vi "Dresden R2R Sputter 03.02.2018 IY24.vi"() -> ()   [LabVIEW 2009] (continued)
                                n24398 = local write "Region"(w29818) -> ()
                                }
                                frame #1 {
                                n24399 = local write "Calculate_auto"(TRUE ("Calculate_auto")) -> ()
                                n24400 = Wait (ms)(milliseconds to wait=u32 1000) -> ()  [unwired: 1 out]
                                }
                                frame #2 {
                                n24401 = local write "Roll_side_select"(enum32{"Left to Right", "Right to Left"}."Left to Right" ("Roll_side_select")) -> ()
                                }
                                frame #3 {
                                n24402 = local write "Parameters_auto_set"(TRUE ("Parameters_auto_set")) -> ()
                                }
                                frame #4 {
                                n24403 = while {
                                i -> [w29834]
                                stop <- w29829 stop-if-true
                                n24404 = Greater?(x=w29834, y=1) -> (0:w29830:bool)
                                n24405 = Wait Until Next ms Multiple(millisecond multiple=u32 300) -> ()  [unwired: 1 out]
                                n24406 = local read "Parameters_auto_set"() -> (w29828:bool)
                                n24407 = case shown="False" w29828 {
                                tunnel: [TRUE FALSE] -> w29831
                                frame #0 {
                                }
                                frame #1 {
                                }
                                }
                                n24408 = Or(x=w29831, y=w29830) -> (x .or. y?=w29829:bool)
                                }
                                }
                                frame #5 {
                                n24409 = local read "R Tension Value"() -> (w29838:dbl)
                                n24410 = Wait (ms)(milliseconds to wait=u32 1000) -> ()  [unwired: 1 out]
                                n24411 = local write "TC1_set_value"(w29838) -> ()
                                }
                                frame #6 {
                                n24412 = local write "TC1_auto_set"(TRUE ("TC1_auto_set")) -> ()
                                }
                                frame #7 {
                                w29840 = u16 0 items=["1", "2", "3", "4"] ("Target Chamber Sensor")
                                n24413 = local write "Target Chamber Sensor"(w29840) -> ()
                                }
                                frame #8 {
                                n24414 = local read "Semi"() -> (w29841:bool)
                                n24415 = case shown="False" w29841 {
                                frame #0 {
                                # "Gas Flow"
                                n24416 = stacked-sequence {
                                frame #0 {
                                n24417 = stacked-sequence {
                                frame #0 {
                                n24418 = local read "Semi"() -> (w29842:bool)
                                n24419 = case shown="False" w29842 {
                                frame #0 {
                                n24420 = local write "Ar_sccm"(u16 200 ("Ar_sccm1_2")) -> ()
                                }
                                frame #1 {
                                }
                                }
                                }
                                frame #1 {
                                n24421 = local read "Semi"() -> (w29844:bool)
                                n24422 = case shown="False" w29844 {
                                frame #0 {
                                n24423 = local write "Mfc_Ar _set"(TRUE ("Mfc_Ar _1_2_set")) -> ()
                                }
                                frame #1 {
                                }
                                }
                                }
                                frame #2 {
                                n24424 = local read "Semi"() -> (w29846:bool)
                                n24425 = case shown="False" w29846 {
                                frame #0 {
                                n24426 = while {
                                i -> [w29850]
                                stop <- w29852 stop-if-true
                                n24427 = Greater?(x=w29850, y=50) -> (0:w29849:bool)
                                n24428 = local read "Semi"() -> (w29848:bool)
                                n24429 = case shown="True" w29848 {
                                tunnel: [FALSE TRUE] -> w29847
                                frame #0 {
                                n24430 = Wait Until Next ms Multiple(millisecond multiple=u32 200) -> ()  [unwired: 1 out]
                                }
                                frame #1 {
                                }
                                }
                                n24431 = Or(x=w29847, y=w29849) -> (x .or. y?=w29852:bool)
                                }
                                }
                                frame #1 {
                                }
                                }
                                }
                                frame #3 {
                                n24432 = local read "Semi"() -> (w29856:bool)
                                n24433 = case shown="False" w29856 {
                                frame #0 {
                                n24434 = local read "Ar_sccm_act 5"() -> (w29858:dbl)
                                n24435 = Greater?(x=w29858, y=1) -> (0:w29857:bool)
                                n24436 = case shown="False" w29857 {
                                frame #0 {
                                n24437 = local write "Ar_sccm"(u16 200 ("Ar_sccm1_2")) -> ()
                                }
                                frame #1 {
                                }
                                }
                                }
                                frame #1 {
                                }
                                }
                                }
                                frame #4 {
                                n24438 = local read "Semi"() -> (w29861:bool)
                                n24439 = case shown="False" w29861 {
                                frame #0 {
                                n24440 = local read "Ar_sccm_act 5"() -> (w29863:dbl)
                                n24441 = Greater?(x=w29863, y=1) -> (0:w29862:bool)
                                n24442 = case shown="False" w29862 {
                                frame #0 {
                                n24443 = while {
                                i -> [w29866]
                                stop <- w29870 stop-if-true
                                n24444 = Greater?(x=w29866, y=50) -> (0:w29865:bool)
                                n24445 = local read "Semi"() -> (w29869:bool)
                                n24446 = case shown="False" w29869 {
                                tunnel: [FALSE TRUE] -> w29868
                                frame #0 {
                                n24447 = Wait Until Next ms Multiple(millisecond multiple=u32 200) -> ()  [unwired: 1 out]
                                }
                                frame #1 {
                                }
                                }
                                n24448 = Or(x=w29868, y=w29865) -> (x .or. y?=w29870:bool)
                                }
                                }
                                frame #1 {
                                }
                                }
                                }
                                frame #1 {
                                }
                                }
                                }
                                frame #5 {
                                n24449 = local read "Semi"() -> (w29874:bool)
                                n24450 = case shown="False" w29874 {
                                frame #0 {
                                n24451 = local read "Ar_sccm_act 5"() -> (w29876:dbl)
                                n24452 = Greater?(x=w29876, y=1) -> (0:w29875:bool)
                                n24453 = case shown="False" w29875 {
                                frame #0 {
                                n24454 = local write "Semi"(TRUE ("Semi")) -> ()
                                n24455 = local write "Error Message"("Coating process cancelled.\nPlease check connections." ("Error Message")) -> ()
                                }
                                frame #1 {
                                }
                                }
                                }
                                frame #1 {
                                }
                                }
                                }
                                }
                                }
                                frame #1 {
                                n24456 = stacked-sequence {
                                frame #0 {
                                n24457 = local read "Semi"() -> (w29880:bool)
                                n24458 = case shown="False" w29880 {
                                frame #0 {
                                n24459 = local read "R_Single Microwave Power"() -> (w29882:dbl)
                                n24460 = Wait (ms)(milliseconds to wait=u32 200) -> ()  [unwired: 1 out]
                                n24461 = local write "Ch1_MW1"(w29882) -> ()
                                }
                                frame #1 {
                                }
                                }
                                }
                                frame #1 {
                                n24462 = local read "Semi"() -> (w29883:bool)
                                n24463 = case shown="False" w29883 {
                                frame #0 {
                                n24464 = local write "Ch1_MW1_set"(TRUE ("Microwave Power_auto_set")) -> ()
                                }
                                frame #1 {
                                }
                                }
                                }
                                frame #2 {
                                n24465 = local read "Semi"() -> (w29885:bool)
                                n24466 = case shown="False" w29885 {
                                frame #0 {
                                n24467 = Wait (ms)(milliseconds to wait=u32 1000) -> ()  [unwired: 1 out]
                                }
                                frame #1 {
                                }
                                }
                                }
                                frame #3 {
                                n24468 = local read "Semi"() -> (w29887:bool)
                                n24469 = case shown="False" w29887 {
                                frame #0 {
                                n24470 = local read "R_Single Microwave Power"() -> (w29889:dbl)
                                n24471 = Wait (ms)(milliseconds to wait=u32 200) -> ()  [unwired: 1 out]
                                n24472 = local write "Ch1_MW2"(w29889) -> ()
                                }
                                frame #1 {
                                }
                                }
                                }
                                frame #4 {
                                n24473 = local read "Semi"() -> (w29890:bool)
                                n24474 = case shown="False" w29890 {
                                frame #0 {
                                n24475 = local write "Ch1_MW2_set"(TRUE ("MW2_Power_set")) -> ()
                                }
                                frame #1 {
                                }
                                }
                                }
                                }
                                }
                                }
                                }
                                frame #1 {
                                }
                                }
                                }
                                frame #9 {
                                n24476 = local write "Start_roll"(TRUE ("Test_auto_start")) -> ()
                                n24477 = Wait (ms)(milliseconds to wait=u32 300) -> ()  [unwired: 1 out]
                                }
                                frame #10 {
                                n24478 = while {
                                stop <- w29895 stop-if-true
                                n24479 = local read "Actual Length"() -> (w29899:dbl)
                                n24480 = local read "Region"() -> (w29898:dbl)
                                n24481 = Greater Or Equal?(x=w29899, y=w29898) -> (x >= y?=w29896:bool)
                                n24482 = local read "Semi"() -> (w29897:bool)
                                n24483 = Or(x=w29896, y=w29897) -> (x .or. y?=w29895:bool)
                                n24484 = Wait Until Next ms Multiple(millisecond multiple=u32 300) -> ()  [unwired: 1 out]
                                }
                                }
                                frame #11 {
                                n24485 = local read "Semi"() -> (w29900:bool)
                                n24486 = case shown="False" w29900 {
                                frame #0 {
                                n24487 = Wait (ms)(milliseconds to wait=u32 1000) -> ()  [unwired: 1 out]
                                n24488 = local write "SMW15"(TRUE ("CMW12")) -> ()
                                }
                                frame #1 {
                                }
                                }
                                }
                                }
                                }
                                frame #1 {
                                }
                                }
                                }
                                frame #2 {
                                n24489 = local read "Semi"() -> (w29903:bool)
                                n24490 = case shown="False" w29903 {
                                frame #0 {
                                n24491 = stacked-sequence {
                                frame #0 {
                                n24492 = local read "R Maximum diameter"() -> (w29908:dbl)
                                n24493 = local read "R Minimum diameter"() -> (w29909:dbl)
                                n24494 = local read "R Web speed(cm/min)"() -> (w29906:dbl)
                                n24495 = local read "R _Total_length"() -> (w29904:dbl)
                                n24496 = local read "R Web thicness"() -> (w29907:dbl)
                                n24497 = Wait (ms)(milliseconds to wait=u32 1000) -> ()  [unwired: 1 out]
                                n24498 = local write "Max Diameter"(w29908) -> ()
                                n24499 = local write "Min Diameter"(w29909) -> ()
                                n24500 = local write "Web Thickness"(w29907) -> ()
                                n24501 = local write "Web Speed"(w29906) -> ()
                                n24502 = local write "Region"(w29904) -> ()
                                }
                                frame #1 {
                                n24503 = local write "Calculate_auto"(TRUE ("Calculate_auto")) -> ()
                                n24504 = Wait (ms)(milliseconds to wait=u32 1000) -> ()  [unwired: 1 out]
                                }
                                frame #2 {
                                n24505 = local write "Roll_side_select"(enum32{"Left to Right", "Right to Left"}."Left to Right" ("Roll_side_select")) -> ()
                                }
                                frame #3 {
                                n24506 = local write "Parameters_auto_set"(TRUE ("Parameters_auto_set")) -> ()
                                }
                                frame #4 {
                                n24507 = while {
                                i -> [w29920]
                                stop <- w29915 stop-if-true
                                n24508 = Greater?(x=w29920, y=100) -> (0:w29916:bool)
                                n24509 = Wait Until Next ms Multiple(millisecond multiple=u32 300) -> ()  [unwired: 1 out]
                                n24510 = local read "Parameters_auto_set"() -> (w29914:bool)
                                n24511 = case shown="False" w29914 {
                                tunnel: [TRUE FALSE] -> w29917
                                frame #0 {
                                }
                                frame #1 {
                                }
                                }
                                n24512 = Or(x=w29917, y=w29916) -> (x .or. y?=w29915:bool)
                                }
                                }
                                frame #5 {
                                n24513 = local read "R Tension Value"() -> (w29924:dbl)
                                n24514 = Wait (ms)(milliseconds to wait=u32 1000) -> ()  [unwired: 1 out]
                                n24515 = local write "TC1_set_value"(w29924) -> ()
                                }
                                frame #6 {
                                n24516 = local write "TC1_auto_set"(TRUE ("TC1_auto_set")) -> ()
                                }
                                frame #7 {
                                w29926 = u16 0 items=["1", "2", "3", "4"] ("Target Chamber Sensor")
                                n24517 = local write "Target Chamber Sensor"(w29926) -> ()
                                }
                                frame #8 {
                                n24518 = local read "Semi"() -> (w29927:bool)
                                n24519 = case shown="False" w29927 {
                                frame #0 {
                                # "Gas Flow"
                                n24520 = stacked-sequence {
                                frame #0 {
                                n24521 = stacked-sequence {
                                frame #0 {
                                n24522 = local read "Semi"() -> (w29928:bool)
                                n24523 = case shown="False" w29928 {
                                frame #0 {
                                n24524 = local write "Ar_sccm"(u16 200 ("Ar_sccm1_2")) -> ()
                                }
                                frame #1 {
                                }
                                }
                                }
                                frame #1 {
                                n24525 = local read "Semi"() -> (w29930:bool)
                                n24526 = case shown="False" w29930 {
                                frame #0 {
                                n24527 = local write "Mfc_Ar _set"(TRUE ("Mfc_Ar _1_2_set")) -> ()
                                }
                                frame #1 {
                                }
                                }
                                }
                                frame #2 {
                                n24528 = local read "Semi"() -> (w29932:bool)
                                n24529 = case shown="False" w29932 {
                                frame #0 {
                                n24530 = while {
                                i -> [w29936]
                                stop <- w29938 stop-if-true
                                n24531 = Greater?(x=w29936, y=50) -> (0:w29935:bool)
                                n24532 = local read "Semi"() -> (w29934:bool)
                                n24533 = case shown="True" w29934 {
                                tunnel: [FALSE TRUE] -> w29933
                                frame #0 {
                                n24534 = Wait Until Next ms Multiple(millisecond multiple=u32 200) -> ()  [unwired: 1 out]
                                }
                                frame #1 {
                                }
                                }
                                n24535 = Or(x=w29933, y=w29935) -> (x .or. y?=w29938:bool)
                                }
                                }
                                frame #1 {
                                }
                                }
                                }
                                frame #3 {
                                n24536 = local read "Semi"() -> (w29942:bool)
                                n24537 = case shown="False" w29942 {
                                frame #0 {
                                n24538 = local read "Ar_sccm_act 5"() -> (w29944:dbl)
                                n24539 = Greater?(x=w29944, y=1) -> (0:w29943:bool)
                                n24540 = case shown="False" w29943 {
                                frame #0 {
                                n24541 = local write "Ar_sccm"(u16 200 ("Ar_sccm1_2")) -> ()
                                }
                                frame #1 {
                                }
                                }
                                }
                                frame #1 {
                                }
                                }
                                }
                                frame #4 {
                                n24542 = local read "Semi"() -> (w29947:bool)
                                n24543 = case shown="False" w29947 {
                                frame #0 {
                                n24544 = local read "Ar_sccm_act 5"() -> (w29949:dbl)
                                n24545 = Greater?(x=w29949, y=1) -> (0:w29948:bool)
                                n24546 = case shown="False" w29948 {
                                frame #0 {
                                n24547 = while {
                                i -> [w29952]
                                stop <- w29956 stop-if-true
                                n24548 = Greater?(x=w29952, y=50) -> (0:w29951:bool)
                                n24549 = local read "Semi"() -> (w29955:bool)
                                n24550 = case shown="False" w29955 {
                                tunnel: [FALSE TRUE] -> w29954
                                frame #0 {
                                n24551 = Wait Until Next ms Multiple(millisecond multiple=u32 200) -> ()  [unwired: 1 out]
                                }
                                frame #1 {
                                }
                                }
                                n24552 = Or(x=w29954, y=w29951) -> (x .or. y?=w29956:bool)
                                }
                                }
                                frame #1 {
                                }
                                }
                                }
                                frame #1 {
                                }
                                }
                                }
                                frame #5 {
                                n24553 = local read "Semi"() -> (w29960:bool)
                                n24554 = case shown="False" w29960 {
                                frame #0 {
                                n24555 = local read "Ar_sccm_act 5"() -> (w29962:dbl)
                                n24556 = Greater?(x=w29962, y=1) -> (0:w29961:bool)
                                n24557 = case shown="False" w29961 {
                                frame #0 {
                                n24558 = local write "Semi"(TRUE ("Semi")) -> ()
                                n24559 = local write "Error Message"("Coating process cancelled.\nPlease check connections." ("Error Message")) -> ()
                                }
                                frame #1 {
                                }
                                }
                                }
                                frame #1 {
                                }
                                }
                                }
                                }
                                }
                                frame #1 {
                                n24560 = stacked-sequence {
                                frame #0 {
                                n24561 = local read "Semi"() -> (w29966:bool)
                                n24562 = case shown="False" w29966 {
                                frame #0 {
                                n24563 = local read "R_Single Microwave Power"() -> (w29968:dbl)
                                n24564 = Wait (ms)(milliseconds to wait=u32 200) -> ()  [unwired: 1 out]
                                n24565 = local write "Ch1_MW1"(w29968) -> ()
                                }
                                frame #1 {
                                }
                                }
                                }
                                frame #1 {
                                n24566 = local read "Semi"() -> (w29969:bool)
                                n24567 = case shown="False" w29969 {
                                frame #0 {
                                n24568 = local write "Ch1_MW1_set"(TRUE ("Microwave Power_auto_set")) -> ()
                                }
                                frame #1 {
                                }
                                }
                                }
                                frame #2 {
                                n24569 = local read "Semi"() -> (w29971:bool)
                                n24570 = case shown="False" w29971 {
                                frame #0 {
                                n24571 = Wait (ms)(milliseconds to wait=u32 1000) -> ()  [unwired: 1 out]
                                }
                                frame #1 {
                                }
                                }
                                }
                                frame #3 {
                                n24572 = local read "Semi"() -> (w29973:bool)
                                n24573 = case shown="False" w29973 {
                                frame #0 {
                                n24574 = local read "R_Single Microwave Power"() -> (w29975:dbl)
                                n24575 = Wait (ms)(milliseconds to wait=u32 200) -> ()  [unwired: 1 out]
                                n24576 = local write "Ch1_MW2"(w29975) -> ()
                                }
                                frame #1 {
                                }
                                }
                                }
                                frame #4 {
                                n24577 = local read "Semi"() -> (w29976:bool)
                                n24578 = case shown="False" w29976 {
                                frame #0 {
                                n24579 = local write "Ch1_MW2_set"(TRUE ("MW2_Power_set")) -> ()
                                }
                                frame #1 {
                                }
                                }
                                }
                                }
                                }
                                }
                                }
                                frame #1 {
                                }
                                }
                                }
                                frame #9 {
                                n24580 = local write "Start_roll"(TRUE ("Test_auto_start")) -> ()
                                n24581 = Wait (ms)(milliseconds to wait=u32 300) -> ()  [unwired: 1 out]
                                }
                                frame #10 {
                                n24582 = while {
                                stop <- w29981 stop-if-true
                                n24583 = local read "Actual Length"() -> (w29985:dbl)
                                n24584 = local read "Region"() -> (w29984:dbl)
                                n24585 = Greater Or Equal?(x=w29985, y=w29984) -> (x >= y?=w29982:bool)
                                n24586 = local read "Semi"() -> (w29983:bool)
                                n24587 = Or(x=w29982, y=w29983) -> (x .or. y?=w29981:bool)
                                n24588 = Wait Until Next ms Multiple(millisecond multiple=u32 300) -> ()  [unwired: 1 out]
                                }
                                }
                                frame #11 {
                                n24589 = stacked-sequence {
                                frame #0 {
                                n24590 = local write "Ch1_MW1"(u16 0 ("Ch1_MW2")) -> ()
                                n24591 = Wait (ms)(milliseconds to wait=u32 1000) -> ()  [unwired: 1 out]
                                }
                                frame #1 {
                                n24592 = local write "Ch1_MW1_set"(TRUE ("Ch1_MW1_set")) -> ()
                                }
                                frame #2 {
                                n24593 = local write "MW1_off"(TRUE ("MW1_off")) -> ()
                                }
                                frame #3 {
                                n24594 = Wait (ms)(milliseconds to wait=u32 1000) -> ()  [unwired: 1 out]
                                }
                                frame #4 {
                                n24595 = local write "Ch1_MW2"(u16 0 ("Ch1_MW2")) -> ()
                                n24596 = Wait (ms)(milliseconds to wait=u32 1000) -> ()  [unwired: 1 out]
                                }
                                frame #5 {
                                n24597 = local write "Ch1_MW2_set"(TRUE ("Ch1_MW2_set")) -> ()
                                }
                                frame #6 {
                                n24598 = local write "MW2_off"(TRUE ("MW2_off")) -> ()
                                }
                                frame #7 {
                                n24599 = local write "SMW20"(TRUE ("CMW16B")) -> ()
                                n24600 = Wait (ms)(milliseconds to wait=u32 1000) -> ()  [unwired: 1 out]
                                }
                                }
                                }
                                frame #12 {
                                n24601 = Wait (ms)(milliseconds to wait=u32 2000) -> ()  [unwired: 1 out]
                                }
                                frame #13 {
                                n24602 = local read "R Maximum diameter"() -> (w30002:dbl)
                                n24603 = local read "R Web speed(cm/min)"() -> (w30000:dbl)
                                n24604 = local read "R Minimum diameter"() -> (w30003:dbl)
                                n24605 = local read "R Web thicness"() -> (w30001:dbl)
                                n24606 = local read "R _Total_length"() -> (w29998:dbl)
                                n24607 = Wait (ms)(milliseconds to wait=u32 1000) -> ()  [unwired: 1 out]
                                n24608 = local write "Max Diameter"(w30002) -> ()
                                n24609 = local write "Web Thickness"(w30001) -> ()
                                n24610 = local write "Min Diameter"(w30003) -> ()
                                n24611 = local write "Web Speed"(w30000) -> ()
                                n24612 = local write "Region"(w29998) -> ()
                                }
                                frame #14 {
                                n24613 = local write "Calculate_auto"(TRUE ("Parameters_auto_set")) -> ()
                                n24614 = Wait (ms)(milliseconds to wait=u32 1000) -> ()  [unwired: 1 out]
                                }
                                frame #15 {
                                n24615 = Wait (ms)(milliseconds to wait=u32 300 ("millisecond multiple")) -> ()  [unwired: 1 out]
                                n24616 = local write "Roll_side_select"(enum32{"Left to Right", "Right to Left"}."Right to Left" ("Roll_side_select")) -> ()
                                }
                                frame #16 {
                                n24617 = local write "Parameters_auto_set"(TRUE ("Parameters_auto_set")) -> ()
                                }
                                frame #17 {
                                n24618 = while {
                                i -> [w30015]
                                stop <- w30010 stop-if-true
                                n24619 = Greater?(x=w30015, y=100) -> (0:w30011:bool)
                                n24620 = Wait Until Next ms Multiple(millisecond multiple=u32 300) -> ()  [unwired: 1 out]
                                n24621 = local read "Parameters_auto_set"() -> (w30009:bool)
                                n24622 = case shown="False" w30009 {
                                tunnel: [TRUE FALSE] -> w30012
                                frame #0 {
                                }
                                frame #1 {
                                }
                                }
                                n24623 = Or(x=w30012, y=w30011) -> (x .or. y?=w30010:bool)
                                }
                                }
                                frame #18 {
                                n24624 = local read "R Tension Value"() -> (w30019:dbl)
                                n24625 = Wait (ms)(milliseconds to wait=u32 1000) -> ()  [unwired: 1 out]
                                n24626 = local write "TC2_set_value"(w30019) -> ()
                                }
                                frame #19 {
                                n24627 = local write "TC2_auto_set"(TRUE ("TC1_auto_set")) -> ()
                                }
                                frame #20 {
                                w30022 = u16 0 items=["1", "2", "3", "4"] ("Target Chamber Sensor")
                                n24628 = local write "Target Chamber Sensor"(w30022) -> ()
                                n24629 = Wait (ms)(milliseconds to wait=u32 1000) -> ()  [unwired: 1 out]
                                }
                                frame #21 {
                                n24630 = Wait (ms)(milliseconds to wait=u32 300) -> ()  [unwired: 1 out]
                                n24631 = local write "Start_roll"(TRUE ("Test_auto_start")) -> ()
                                }
                                frame #22 {
                                n24632 = stacked-sequence {
                                frame #0 {
                                n24633 = local read "Semi"() -> (w30025:bool)
                                n24634 = case shown="False" w30025 {
                                frame #0 {
                                n24635 = local read "R_Single Microwave Power"() -> (w30027:dbl)
                                n24636 = Wait (ms)(milliseconds to wait=u32 200) -> ()  [unwired: 1 out]
                                n24637 = local write "Ch1_MW1"(w30027) -> ()
                                }
                                frame #1 {
                                }
                                }
                                }
                                frame #1 {
                                n24638 = local read "Semi"() -> (w30028:bool)
                                n24639 = case shown="False" w30028 {
                                frame #0 {
                                n24640 = local write "Ch1_MW1_set"(TRUE ("Microwave Power_auto_set")) -> ()
                                }
                                frame #1 {
                                }
                                }
                                }
                                frame #2 {
                                n24641 = local read "Semi"() -> (w30030:bool)
                                n24642 = case shown="False" w30030 {
                                frame #0 {
                                n24643 = Wait (ms)(milliseconds to wait=u32 1000) -> ()  [unwired: 1 out]
                                }
                                frame #1 {
                                }
                                }
                                }
                                frame #3 {
                                n24644 = local read "Semi"() -> (w30032:bool)
                                n24645 = case shown="False" w30032 {
                                frame #0 {
                                n24646 = local read "R_Single Microwave Power"() -> (w30034:dbl)
                                n24647 = Wait (ms)(milliseconds to wait=u32 200) -> ()  [unwired: 1 out]
                                n24648 = local write "Ch1_MW2"(w30034) -> ()
                                }
                                frame #1 {
                                }
                                }
                                }
                                frame #4 {
                                n24649 = local read "Semi"() -> (w30035:bool)
                                n24650 = case shown="False" w30035 {
                                frame #0 {
                                n24651 = local write "Ch1_MW2_set"(TRUE ("MW2_Power_set")) -> ()
                                }
                                frame #1 {
                                }
                                }
                                }
                                }
                                }
                                frame #23 {
                                n24652 = while {
                                stop <- w30037 stop-if-true
                                n24653 = local read "Actual Length"() -> (w30042:dbl)
                                n24654 = local read "Region"() -> (w30041:dbl)
                                n24655 = Greater Or Equal?(x=w30042, y=w30041) -> (x >= y?=w30039:bool)
                                n24656 = local read "Semi"() -> (w30040:bool)
                                n24657 = Or(x=w30039, y=w30040) -> (x .or. y?=w30037:bool)
                                n24658 = Wait Until Next ms Multiple(millisecond multiple=u32 300) -> ()  [unwired: 1 out]
                                }
                                }
                                frame #24 {
                                n24659 = local read "Semi"() -> (w30043:bool)
                                n24660 = case shown="False" w30043 {
                                frame #0 {
                                n24661 = Wait (ms)(milliseconds to wait=u32 1000) -> ()  [unwired: 1 out]
                                n24662 = local write "SMW15"(TRUE ("CMW12")) -> ()
                                }
                                frame #1 {
                                }
                                }
                                }
                                }
                                }
                                frame #1 {
                                }
                                }
                                }
                                }
                                }
                                }
                                }
                                frame #14 {
                                # "CLOSE MW"
                                n24663 = local read "Semi"() -> (w30046:bool)
                                n24664 = case shown="False" w30046 {
                                frame #0 {
                                n24665 = stacked-sequence {
                                frame #0 {
                                n24666 = local write "Ch1_MW1"(u16 0 ("Ch1_MW2")) -> ()
                                n24667 = Wait (ms)(milliseconds to wait=u32 1000) -> ()  [unwired: 1 out]
                                }
                                frame #1 {
                                n24668 = local write "Ch1_MW1_set"(TRUE ("Ch1_MW1_set")) -> ()
                                }
                                frame #2 {
                                n24669 = local write "MW1_off"(TRUE ("MW1_off")) -> ()
                                }
                                frame #3 {
                                n24670 = Wait (ms)(milliseconds to wait=u32 1000) -> ()  [unwired: 1 out]
                                }
                                frame #4 {
                                n24671 = local write "Ch1_MW2"(u16 0 ("Ch1_MW2")) -> ()
                                n24672 = Wait (ms)(milliseconds to wait=u32 1000) -> ()  [unwired: 1 out]
                                }
                                frame #5 {
                                n24673 = local write "Ch1_MW2_set"(TRUE ("Ch1_MW2_set")) -> ()
                                }
                                frame #6 {
                                n24674 = local write "MW2_off"(TRUE ("MW2_off")) -> ()
                                }
                                frame #7 {
                                n24675 = local write "SMW20"(TRUE ("CMW16B")) -> ()
                                n24676 = Wait (ms)(milliseconds to wait=u32 1000) -> ()  [unwired: 1 out]
                                }
                                }
                                }
                                frame #1 {
                                }
                                }
                                }
                                frame #15 {
                                # "PC-BV OPEN"
                                n24677 = stacked-sequence {
                                frame #0 {
                                n24678 = local read "Semi"() -> (w30058:bool)
                                n24679 = case shown="False" w30058 {
                                frame #0 {
                                n24680 = stacked-sequence {
                                frame #0 {
                                n24681 = local read "Semi"() -> (w30059:bool)
                                n24682 = case shown="False" w30059 {
                                frame #0 {
                                n24683 = local write "Pc_bv1_auto_open"(TRUE ("Tp1_auto_start")) -> ()
                                }
                                frame #1 {
                                }
                                }
                                }
                                frame #1 {
                                n24684 = local read "Semi"() -> (w30061:bool)
                                n24685 = case shown="False" w30061 {
                                frame #0 {
                                n24686 = Wait (ms)(milliseconds to wait=u32 1000) -> ()  [unwired: 1 out]
                                }
                                frame #1 {
                                }
                                }
                                }
                                frame #2 {
                                n24687 = local read "Semi"() -> (w30063:bool)
                                n24688 = case shown="False" w30063 {
                                frame #0 {
                                n24689 = while {
                                i -> [w30069]
                                stop <- w30065 stop-if-true
                                n24690 = local read "Pc_bv_opened_ch1"() -> (w30067:bool)
                                n24691 = Greater?(x=w30069, y=120) -> (0:w30068:bool)
                                n24692 = local read "Semi"() -> (w30066:bool)
                                n24693 = Compound Arithmetic op=OR(w30066, w30067, w30068) -> (w30065:bool)
                                n24694 = Wait (ms)(milliseconds to wait=u32 500) -> ()  [unwired: 1 out]
                                }
                                }
                                frame #1 {
                                }
                                }
                                }
                                frame #3 {
                                n24695 = local read "Semi"() -> (w30071:bool)
                                n24696 = case shown="False" w30071 {
                                frame #0 {
                                n24697 = local read "Pc_bv_opened_ch1"() -> (w30072:bool)
                                n24698 = case shown="False" w30072 {